vi "ContinousCameraStageV2.vi"() -> ()   [LabVIEW 2016]
uses:
  <vilib>/userdefined/High Color/IMAQdx.ctl
  Controls/0_XYZstage/DoHomeControl.ctl
  Controls/0_XYZstage/JogControlPanel.ctl
  Controls/All_Enums/Enum_TypeDef_JogStepSize.ctl
  Controls/0_XYZstage/CurrentPositionReader.ctl
  Controls/0_XYZstage/BOOLs_AxesEnabled.ctl
  Controls/0_XYZstage/CurrentMonitoring.ctl
  Controls/0_XYZstage/BOOL_Moving.ctl
  Controls/All_Enums/Enum_TypeDef_ImageSharpnessAnalysisMethod.ctl
  Controls/Graph_TypeDef_XY.ctl
  <vilib>/vision/Image Controls.llb/IMAQ Image.ctl
  AerotechLibraries/Motion/MoveIncMultiple.vi
  AerotechLibraries/Motion/WaitMultiple.vi
  <vilib>/vision/driver/NI_Vision_Acquisition_Software.lvlib
  <vilib>/vision/NI_Vision_Development_Module.lvlib
  <vilib>/LabVIEW Interface for Arduino/LabVIEW Interface for Arduino.lvlib
panel:
  out "Z [mm]":dbl
  in  "Tab Control":T1(tab)
  in  "Tab Control 2":enum32{"Stage Controls", "Camera Controls"}(tab)
  in  "Save current position":bool
  in  "Move Stage with Cursors":bool
  in  "Home stage?":T2
  in  "Jogging Controls":T3={"Jog step size"={"X [mm]"=enum."1 mm", "Y [mm]"=enum."1 mm", "Z [mm]"=enum."1 mm"}, "Left"=FALSE, "Right"=FALSE, "Forward"=FALSE, "Backward"=FALSE, "Up"=FALSE, "Down"=FALSE, "Reset position"=FALSE, "Confirm position"=FALSE}
  in  "Axes Speeds":T5={"X [mm/s]"=25.0, "Y [mm/s]"=25.0, "Z [mm/s]"=25.0}
  in  "Move to Absolute Position [mm]":T6
  in  "Move Stage":bool
  out "Cross Point":cluster{"X coordinate":dbl, "Y coordinate":dbl}
  in  "Abort stage":bool
  in  "Tab Control 4":T7(tab)
  in  "Camera Name":T8="cam1" caption="IMAQdx Session"
  in  "Wait time before \nimage capture [s]":dbl=3.5
  in  "Gain of the Camera":dbl(slide) scale=0.0..16.0
  out "Intensity Histogram, current frame":T9(graph)
  in  "Pixel to Micron":dbl=1.5810615417510199 format="%.4f"
  in  "Conversion Method":u16(ring)=1 items=["Strip Centers", "Signal Fit, Left to Right", "Projection + Signal Fit"]
  out "Skew Angle [radians]":dbl format="%.5f"
  out "Skew Angle (uncertainty)":dbl format="%.5f"
  out "um/pixel uncertainty":dbl format="%.4f"
  in  "Strips Coordinates":T6={"X [mm]"=-738.0, "Y [mm]"=-144.0, "Z [mm]"=34.25}
  in  "Strip Pitch (microns)":dbl=74.5 format="%#_13g"
  out "Optimized position":dbl
  out "Uncertainty on position":dbl
  in  "Camera working distance scan":T10={"Stepsize [mm]"=0.2, "Focusing test interval [mm]"=1.5} {"Focusing test interval [mm]" format="%#_13g"}
  in  "Method":T11
  out "Plot":T12
  out "Autofocus Progress":u8(slide) scale=0.0..15.0
  in  "Settings":T13={"Algorithm"=1, "Number of Matches Requested"=1, "Minimum Match Score"=700.0, "SubPixel Accuracy"=TRUE, "Rotation Angle Ranges"=[{"Start"=0.0, "End"=360.0}], "Show Search Area"=FALSE, "Show Result"=TRUE} {"Rotation Angle Ranges"."End" format="%.1f"; "Rotation Angle Ranges"."Start" format="%.1f"; "Minimum Match Score" min=0 max=1000 format="%.2f"; "Number of Matches Requested" min=1; "Algorithm" items=["All", "Low Discrepancy Sampling", "Grayscale Value Pyramid", "Gradients Pyramid"]}
  out "1st Match Distance from Center":cluster{dbl, dbl}
  in  "Template Path":path
  out "1st Matched Position":cluster{"X":dbl, "Y":dbl, "Z [mm]":dbl}
  out "Template Image":T14(plugin-control)
  out "Eccentricity vs. Threshold":cluster{i32[], dbl[]}(graph)
  in  "Threshold Max":sgl=255.0
  in  "Primary Light":bool
  in  "Camera Analysis Function":T15(ring)
  in  "Spotlights":bool
  out "Current stage position":T16
  out "Current monitoring":T17
  out "Homed":bool
  out "Moving":T18
  out "Axis enabled":T19
  out "Wait to capture [ms]":u32=3500
  in  "X [mm]":dbl(slide)=5.417536534446764 scale=-1.0..6.596742723794349 scale format="%#_3g"
  in  "Y [mm]":dbl(slide)=4.6938775510204085 scale=4.720794011715331..-1.0 scale format="%#_3g"
  in  "Tab Control 3":T20(tab)
  out "Current field of view":T14(plugin-control)
  out "Bullseye Out":T14(plugin-control)
  out "Ellipses Out":T14(plugin-control)
  in  "Click to Stop The Program":bool
  out "double( Time, Temp )":dbl[](array[numeric])=[14.0, 16.0, 34.0, 0.8858232498168945, 22.9537926]
  in  "Program Errors 2":errorcluster
  in  "Program Errors":errorcluster
  out "VISA error out":errorcluster
  out "Camera error out":errorcluster
  out "Time and Temperature [*C]":string[](array[string])
  # "CONTINUOUS STAGE AND CAMERA (v2) Brandeis University - Brookhaven National Laboratory * ATLAS Phase II Inner Tracker Upgrade\nPrimary Authors: Prajita Bhattarai (pbhattarai1s@brandeis.edu), Hannah Herde (hherde@brandeis.edu)"
  # "XYZ Stage Performance Monitoring"
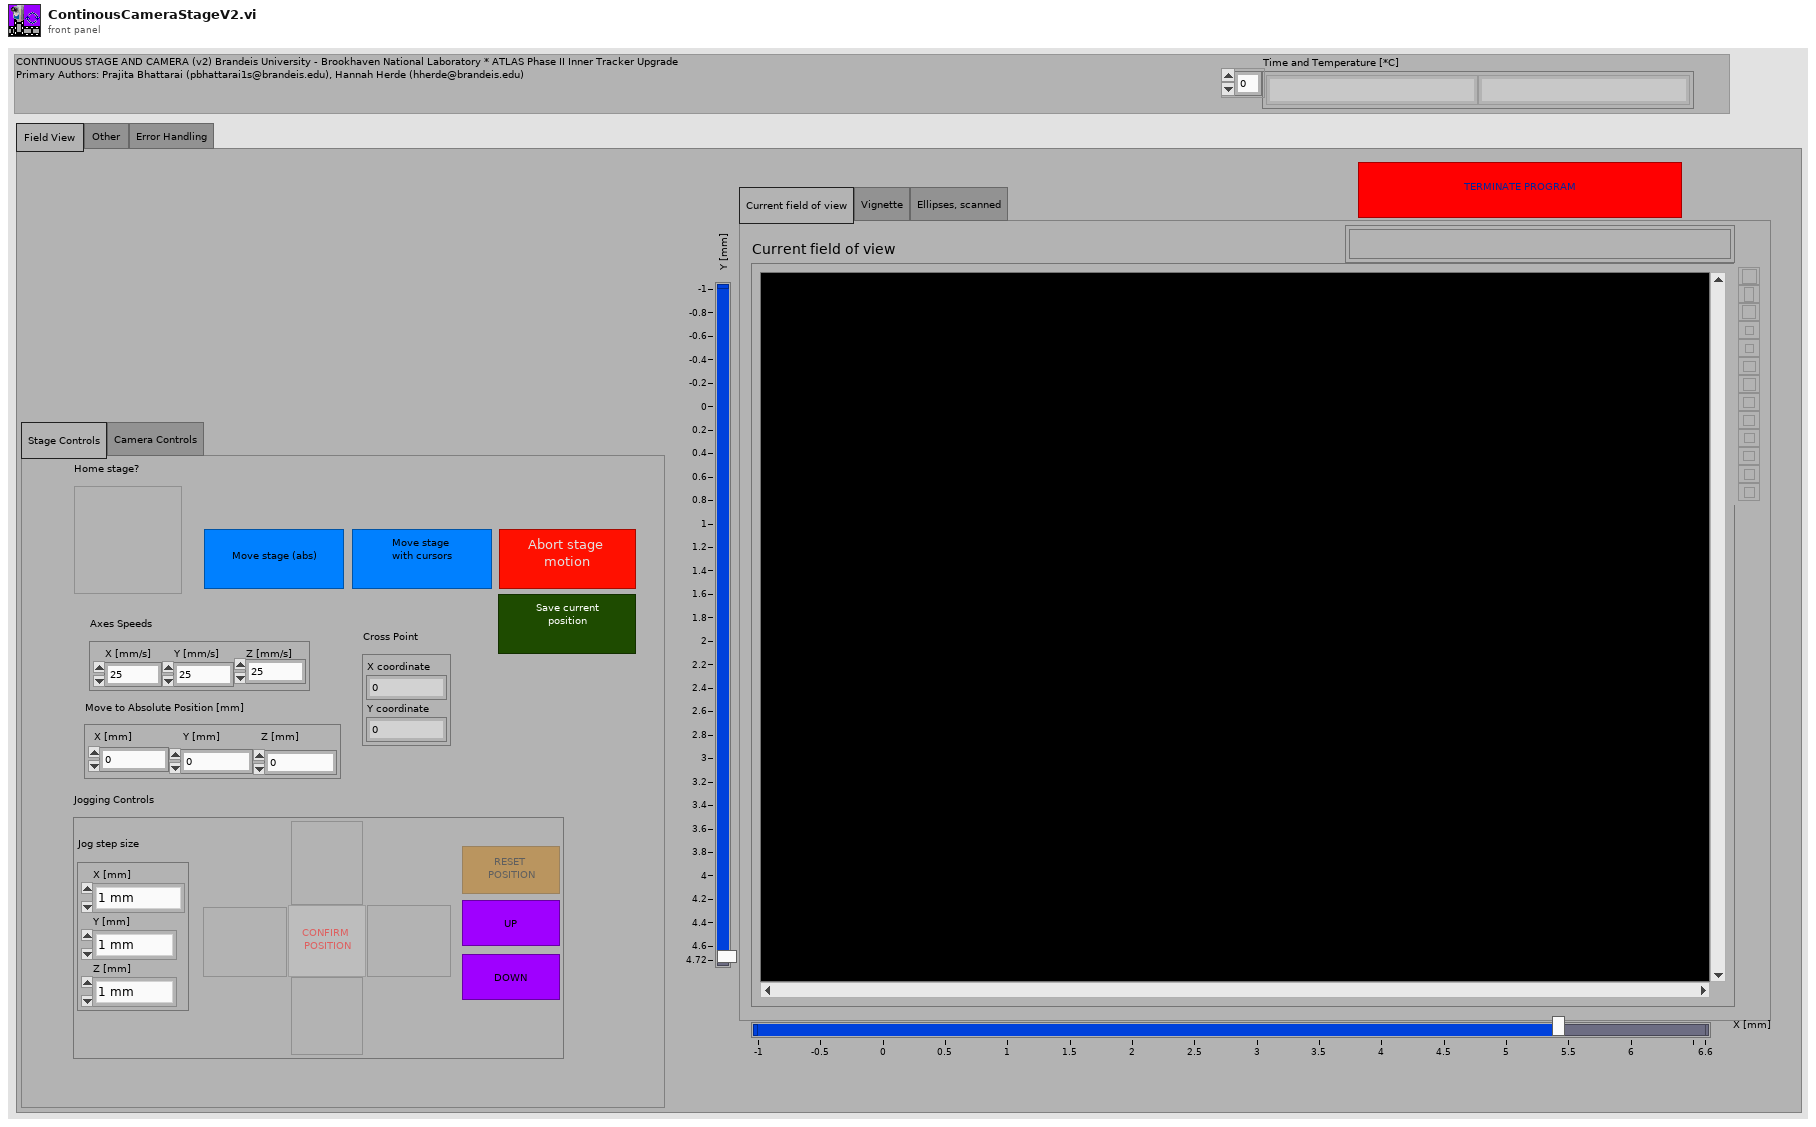
[diagram p1: front panel]
types:
  T1 = enum32{"Field View ", "Other ", "Error Handling"}
  T2 = typedef "DoHomeControl.ctl" = bool
  T3 = typedef "JogControlPanel.ctl" = cluster{"Jog step size":T4, "Left":bool, "Right":bool, "Forward":bool, "Backward":bool, "Up":bool, "Down":bool, "Reset position":bool, "Confirm position":bool}
  T4 = typedef "Enum_TypeDef_JogStepSize.ctl" = cluster{"X [mm]":enum16{"1 um", "5 um", "10 um", "0.1 mm", "0.25 mm", "0.5 mm", "1 mm", "5 mm", "10 mm", "20 mm", "50 mm"}, "Y [mm]":enum16{"1 um", "5 um", "10 um", "0.1 mm", "0.25 mm", "0.5 mm", "1 mm", "5 mm", "10 mm", "20 mm", "50 mm"}, "Z [mm]":enum16{"1 um", "5 um", "10 um", "0.1 mm", "0.25 mm", "0.5 mm", "1 mm", "5 mm", "10 mm", "20 mm", "[None]"}}
  T5 = cluster{"X [mm/s]":dbl, "Y [mm/s]":dbl, "Z [mm/s]":dbl}
  T6 = cluster{"X [mm]":dbl, "Y [mm]":dbl, "Z [mm]":dbl}
  T7 = enum32{"Camera Setup", "Pixel/Micron Conv.", "Height/Autofocus", "Pattern Match", "Vignetting Analysis"}
  T8 = typedef "IMAQdx.ctl" = refnum<k21>
  T9 = cluster{"Starting Value":sgl, "Incremental Value":sgl, "Histogram":u32[]}
  T10 = cluster{"Stepsize [mm]":dbl, "Focusing test interval [mm]":dbl}
  T11 = typedef "Enum_TypeDef_ImageSharpnessAnalysisMethod.ctl" = enum16{"sigma( Intensity )", "Mean( Laplacian Convolution )"}
  T12 = typedef "Graph_TypeDef_XY.ctl" = cluster{"Radius bins":dbl[], "Best Gaussian Fit":dbl[]}[]
  T13 = cluster{"Algorithm":i32, "Number of Matches Requested":i32, "Minimum Match Score":sgl, "SubPixel Accuracy":bool, "Rotation Angle Ranges":cluster{"Start":sgl, "End":sgl}[], "Show Search Area":bool, "Show Result":bool}
  T14 = typedef "IMAQ Image.ctl" = refnum<image>
  T15 = enum16{"[None]", "Determine pixel-micron conversion", "Calibrate camera height", "Find a pattern", "Analyze vignette"}
  T16 = typedef "CurrentPositionReader.ctl" = cluster{"X":dbl, "Y":dbl, "Z":dbl}
  T17 = typedef "CurrentMonitoring.ctl" = cluster{cluster{"X Current Cmd [A]":sgl, "Y Current Cmd [A]":sgl, "Z Current Cmd [A]":sgl}, cluster{"X Current Feedback [A]":sgl, "Y Current Feedback [A]":sgl, "Z Current Feedback [A]":sgl}}
  T18 = typedef "BOOL_Moving.ctl" = bool
  T19 = typedef "BOOLs_AxesEnabled.ctl" = cluster{"X":bool, "Y ":bool, "Z":bool}
  T20 = enum32{"Current field of view", "Vignette", "Ellipses, scanned"}
  T21 = typedef "Image Type" = u32
  T22 = typedef "LabVIEW Interface for Arduino.lvlib/Arduino Resource.ctl" = cluster{"VISA resource":refnum<visa-resource-name>, "Board Type":T23, "Connection Type":enum8{"USB / Serial"}, "Bytes Per Packet (15)":u8}
  T23 = typedef "LabVIEW Interface for Arduino.lvlib/Board Type.ctl" = enum16{"Uno", "Dimuelanove w/Atmega 328", "Mega 2560"}
  T24 = typedef "ArduinoLT-ConfigurationControl.ctl" = cluster{"Lights: Digital I/O Pins":cluster{"Coaxial":u8, "Spotlights":u8}, "Thermistor Settings":cluster{"Analogue Readout Pin":u8, "Vcc Reference Pin":u8, "Paired Resistance (10K Ohms)":dbl, "Units (C)":enum16{"Celsius", "Fahrenheit", "Kelvin"}}}
  T25 = cluster{"Camera session out":T8, "New Image":T14}
  T26 = cluster{"Final X":dbl, "Final Y":dbl, "Final Z":dbl}
  T27 = cluster{"X":dbl, "Y":dbl, "Optimized position":dbl}
  T28 = cluster{"Position":cluster{"x":sgl, "y":sgl}, "Angle":sgl, "Scale":sgl, "Score":sgl, "Bounding Box":cluster{"x":sgl, "y":sgl}[]}[]
  T29 = cluster{"Matches (pixel)[0]":cluster{"Position":cluster{"x":sgl, "y":sgl}, "Angle":sgl, "Scale":sgl, "Score":sgl, "Bounding Box":cluster{"x":sgl, "y":sgl}[]}, "Matches (pixel)[1]":cluster{"Position":cluster{"x":sgl, "y":sgl}, "Angle":sgl, "Scale":sgl, "Score":sgl, "Bounding Box":cluster{"x":sgl, "y":sgl}[]}, "Matches (pixel)[2]":cluster{"Position":cluster{"x":sgl, "y":sgl}, "Angle":sgl, "Scale":sgl, "Score":sgl, "Bounding Box":cluster{"x":sgl, "y":sgl}[]}, "Matches (pixel)[3]":cluster{"Position":cluster{"x":sgl, "y":sgl}, "Angle":sgl, "Scale":sgl, "Score":sgl, "Bounding Box":cluster{"x":sgl, "y":sgl}[]}, "Matches (pixel)[4]":cluster{"Position":cluster{"x":sgl, "y":sgl}, "Angle":sgl, "Scale":sgl, "Score":sgl, "Bounding Box":cluster{"x":sgl, "y":sgl}[]}, "Matches (pixel)[5]":cluster{"Position":cluster{"x":sgl, "y":sgl}, "Angle":sgl, "Scale":sgl, "Score":sgl, "Bounding Box":cluster{"x":sgl, "y":sgl}[]}, "Matches (pixel)[6]":cluster{"Position":cluster{"x":sgl, "y":sgl}, "Angle":sgl, "Scale":sgl, "Score":sgl, "Bounding Box":cluster{"x":sgl, "y":sgl}[]}, "Matches (pixel)[7]":cluster{"Position":cluster{"x":sgl, "y":sgl}, "Angle":sgl, "Scale":sgl, "Score":sgl, "Bounding Box":cluster{"x":sgl, "y":sgl}[]}, "Matches (pixel)[8]":cluster{"Position":cluster{"x":sgl, "y":sgl}, "Angle":sgl, "Scale":sgl, "Score":sgl, "Bounding Box":cluster{"x":sgl, "y":sgl}[]}}
  T30 = cluster{"Position":cluster{"x":sgl, "y":sgl}, "Angle":sgl, "Scale":sgl, "Score":sgl, "Bounding Box":cluster{"x":sgl, "y":sgl}[]}
  T31 = cluster{cluster{"X Current Cmd [A]":sgl, "Y Current Cmd [A]":sgl, "Z Current Cmd [A]":sgl}, cluster{"X Current Feedback [A]":sgl, "Y Current Feedback [A]":sgl, "Z Current Feedback [A]":sgl}}
  T32 = cluster{"Step size [mm]":dbl, "Step size [mm]":dbl, "Step size [mm]":dbl}
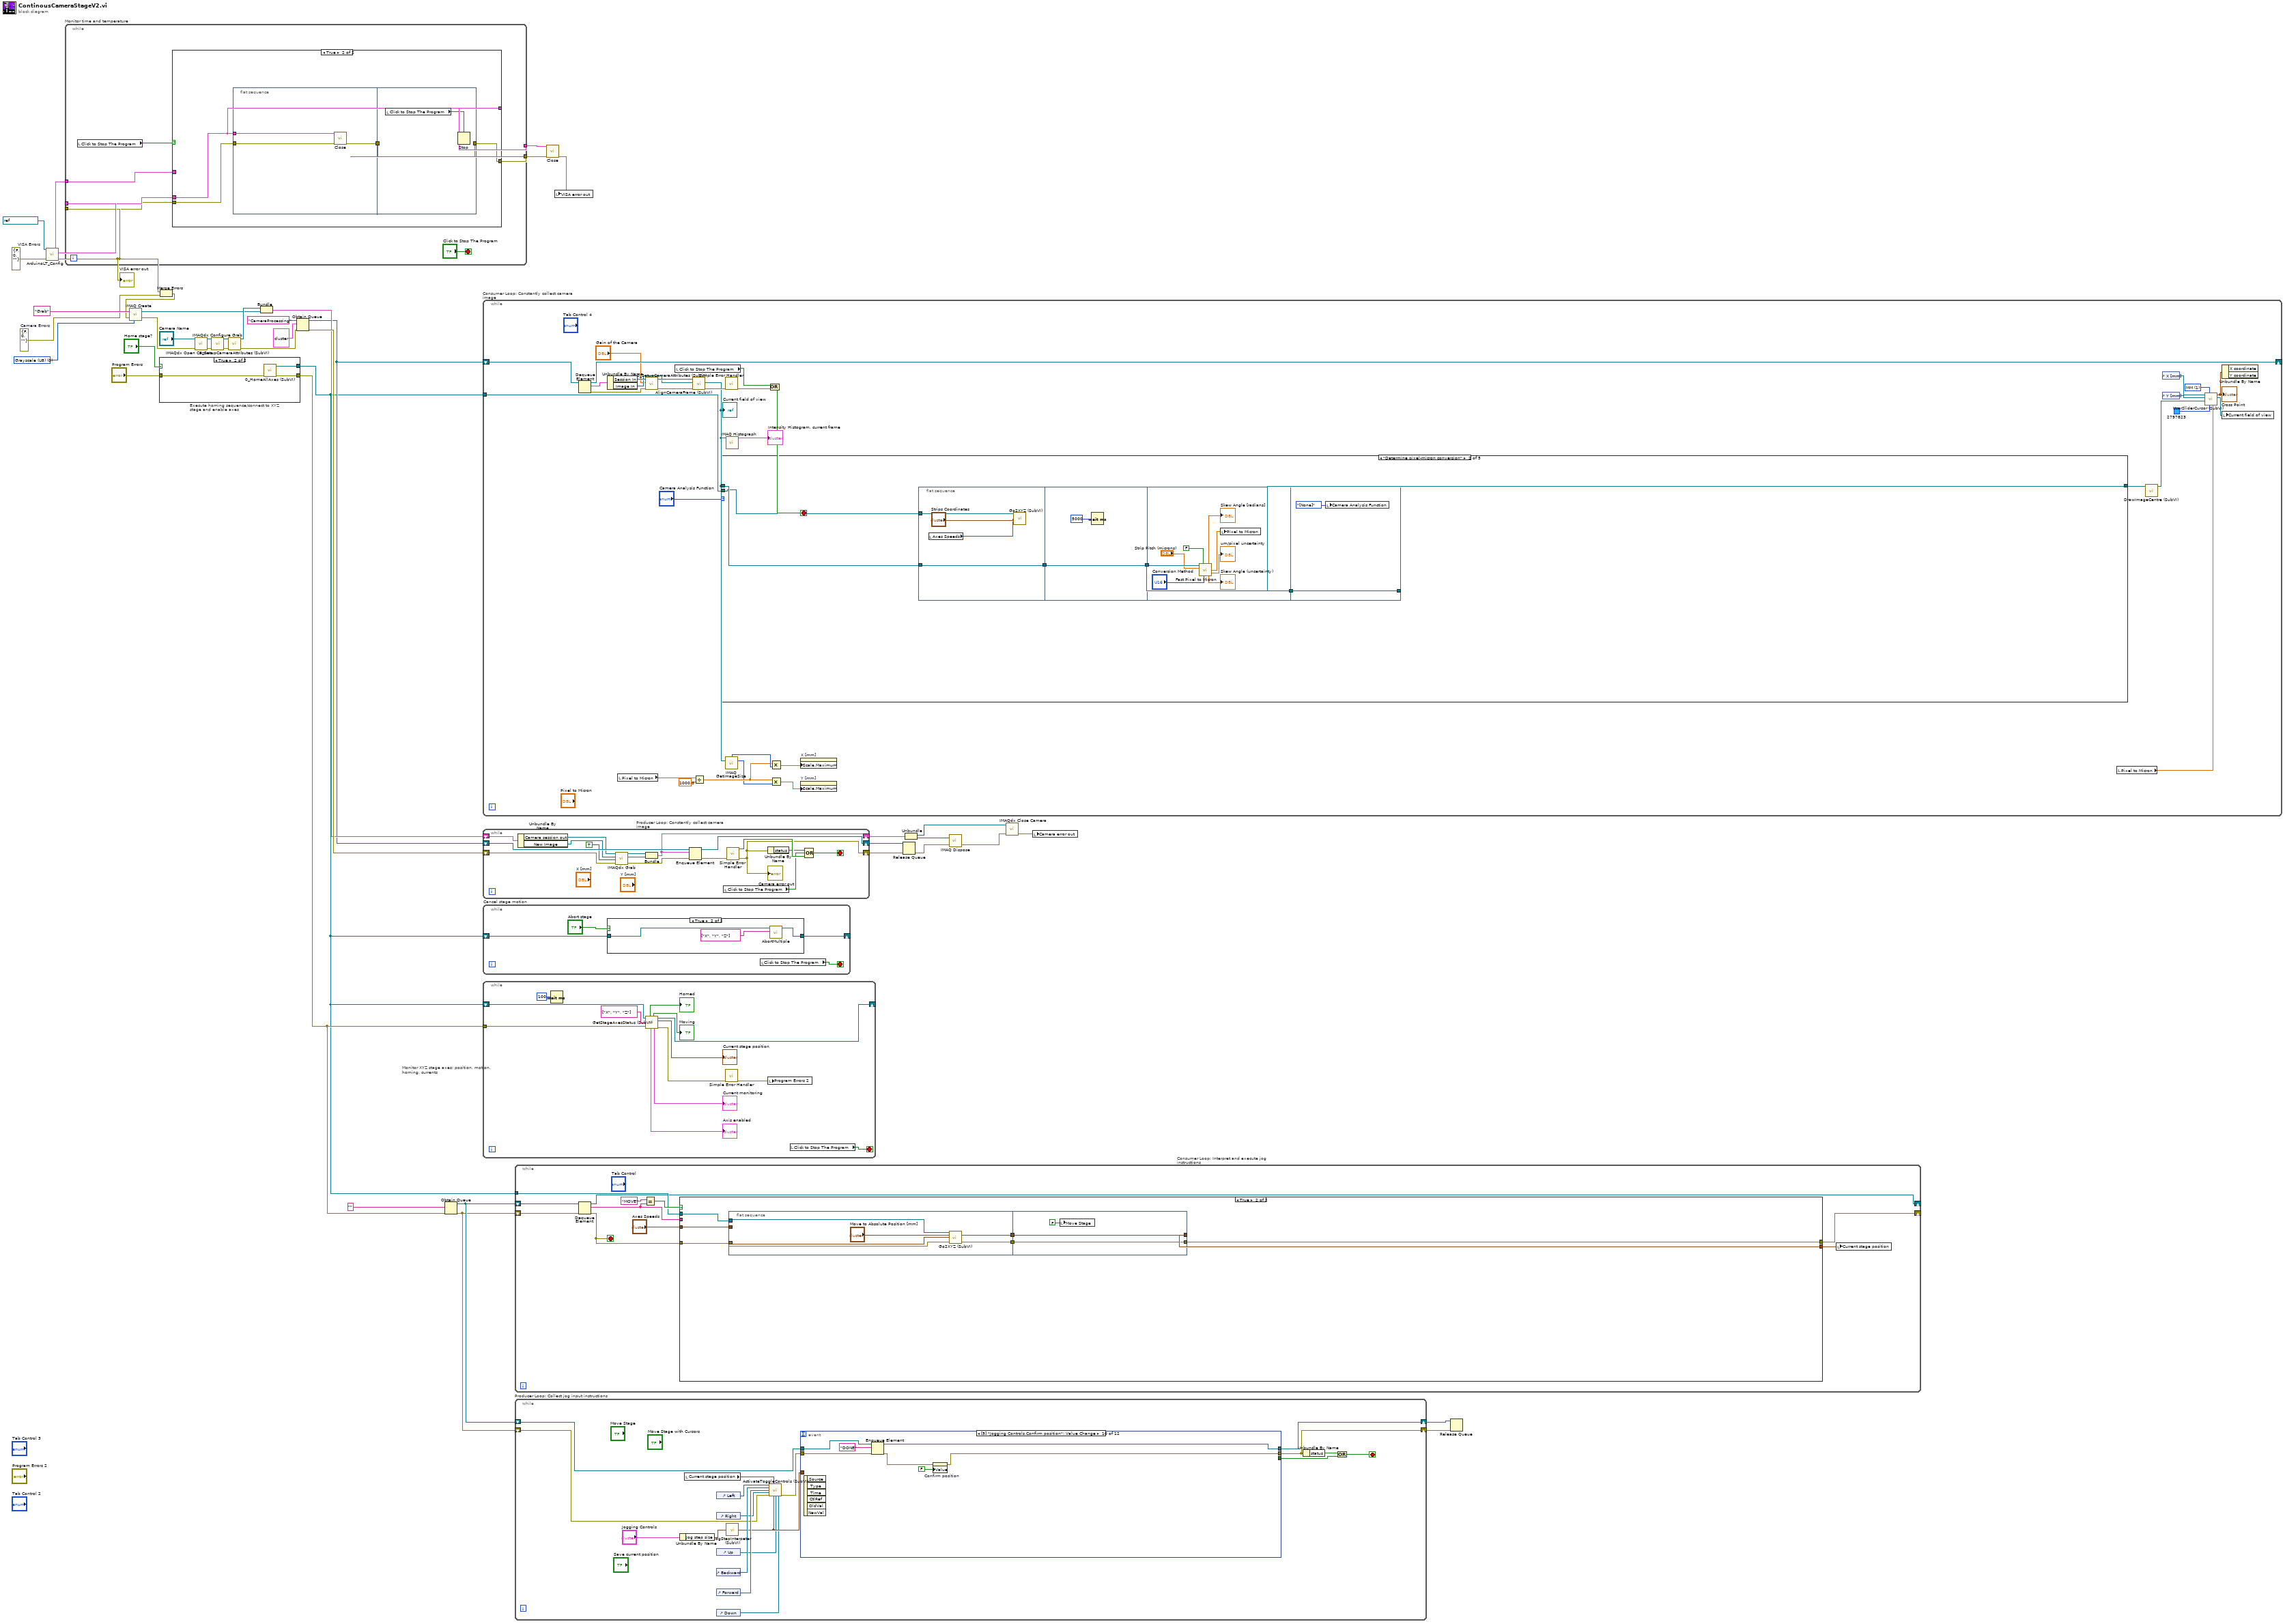
[diagram p0: block diagram]
diagram:
  w9 = errorcluster {"status"=FALSE, "code"=0, "source"=""}  # VISA Errors
  w2 = errorcluster {"status"=FALSE, "code"=0, "source"=""}  # Camera Errors
  w41 = T21 0 items=["Grayscale (U8)", "Grayscale (I16)", "Grayscale (SGL)", "Complex (CSG)", "RGB (U32)", "HSL (U32)", "RGB (U64)", "Grayscale (U16)"] ("Image Type")
  n1 = call "ArduinoLT_Config.vi"("error in"=w9, "VISA resource"=refnum<visa-resource-name> "LightsCTRL") -> ("error out"=w3:errorcluster, "Arduino Resource"=w7:T22, "Arduino Configuration OUT"=w8:T24)  [unwired: 3 in, 1 out]
  "VISA error out" <- w3
  n2 = while "Monitor time and temperature" {
    tunnel: w3 -> [w47]
    tunnel: w8 -> [w49]
    tunnel: w7 -> [w48]
    tunnel: [w46] -> w6
    tunnel: [w45] -> w4
    stop <- "Click to Stop The Program" stop-if-true
    n3 = local read "Click to Stop The Program"() -> (w44:bool)
    n4 = case shown="True" w44 {
      tunnel: w49 -> [w59 _]
      tunnel: w48 -> [w58 w66]
      tunnel: w47 -> [w57 w69]
      tunnel: [w56 w66] -> w46
      tunnel: [w52 w68] -> w45
      frame False {
        n5 = Wait (ms)(milliseconds to wait=u32 1000) -> ()  [unwired: 1 out]
        n6 = call "ArduinoLT_Collect_Control.vi"("Arduino Configuration"=w59, "error in"=w57, "Arduino Resource IN"=w58, "Spotlights"="Spotlights", "Coaxial light"="Primary Light") -> ("error out"=w51:errorcluster, "Arduino Resource OUT"=w56:T22, "Thermometer [C]"=w55:dbl)  [unwired: 4 in]
        n7 = local write "VISA error out"(w51) -> ()
        n8 = Multiply(x="Wait time before \nimage capture [s]", y=u32 1000) -> (x*y=→"Wait to capture [ms]":dbl)
        n9 = call "ArduinoLT-TimeAndTempature.vi"("error in (no error)"=w51, "Temperature"=w55) -> ("error out"=w52:errorcluster, "double( Time, Temp )"=→"double( Time, Temp )":dbl[], "str( Time, Temp )"=→"Time and Temperature [*C]":string[])  [unwired: 7 in]
        n10 = local write "VISA error out"(w52) -> ()
      }
      frame True {
        n11 = flat-sequence {
          tunnel: w66 -> [w72]
          tunnel: w69 -> [w71]
          tunnel: [w70] -> w67
          tunnel: [w74] -> w68
          tunnel: w67 -> [w74]
          frame #0 {
            n12 = call <vilib>:"Close.vi"("Arduino Resource"=w72, "error in"=w71) -> ("error out"=w70:errorcluster)  [unwired: 13 in]
          }
          frame #1 {
            n13 = local read "Click to Stop The Program"() -> (w73:bool)
            n14 = Stop(stop? (T)=w73) -> ()
          }
        }
      }
    }
  }
  n15 = case "Execute homing sequence/connect to XYZ stage and enable axes" shown="True" "Home stage?" {
    tunnel: [w77 w83] -> w12
    tunnel: "Program Errors" -> [w75 w81]
    tunnel: [w76 w82] -> w11
    frame False {
      n16 = call "Connect.vi"("error in (no error)"=w75) -> ("error out"=w80:errorcluster, "controller"=w79:refnum<k24>)  [unwired: 9 in]
      n17 = call "EnableMultiple.vi"("error in (no error)"=w80, "axis names"=string[] ["X", "Y", "Z"] ("Axes Names"), "controller in"=w79) -> ("error out"=w77:errorcluster, "controller out"=w76:refnum<k24>)  [unwired: 7 in]
    }
    frame True {
      n18 = call "0_HomeAllAxes (SubVI).vi"("error in (no error)"=w81) -> ("error out"=w83:errorcluster, "controller out"=w82:refnum<k24>)  [unwired: 7 in, 2 out]
    }
  }
  n19 = Merge Errors(w3, w2) -> (w1:errorcluster)
  n20 = call "IMAQ Create"("Image Name"="Grab", "Image Type"=w41, "error in (no error)"=w1) -> ("New Image"=w30:T14, "error out"=w38:errorcluster)  [unwired: 1 in, 1 out]
  n21 = call <vilib>:"IMAQdx Open Camera.vi"("error in"=w38, "Session In"="Camera Name") -> ("error out"=w39:errorcluster, "Session Out"=w42:T8)  [unwired: 1 in, 7 out]
  n22 = call <vilib>:"IMAQdx Configure Grab.vi"("error in"=w39, "Session In"=w42) -> ("error out"=w34:errorcluster, "Session Out"=w35:T8)  [unwired: 8 out]
  n23 = call "0_SetupCameraAttributes (SubVI).vi"("error in (no error)"=w34, "Camera session in"=w35) -> ("error out"=w33:errorcluster, "Camera session out"=w31:T8)  [unwired: 8 in]
  n24 = Bundle("Camera session out"=w31, "New Image"=w30) -> (w29:T25)  [unwired: 1 in]
  n25 = Obtain Queue(name (unnamed)="CameraProcessing", element data type=cluster{"Session In":T8, "Image In":T14} {"Session In"="", "Image In"=refnum}, error in (no error)=w33) -> (queue out=w21:refnum<queue>, error out=w32:errorcluster)  [unwired: 2 in, 1 out]
  n26 = Obtain Queue(element data type="", error in (no error)=w12) -> (queue out=w16:refnum<queue>, error out=w15:errorcluster)  [unwired: 3 in, 1 out]
  n27 = while "Consumer Loop: Constantly collect camera image" {
    shift-right: [w112] -> _
    shift-left: w21 -> [w116]
    tunnel: w11 -> [w99]
    stop <- w114 stop-if-true
    w89 = u16 1 items=["MM"=1, "Pixel"=0] ("Coordinates Unit")
    n28 = Dequeue Element(queue=w116) -> (queue out=w112:refnum<queue>, element=w115:cluster{"Session In":T8, "Image In":T14}, error out=w113:errorcluster)  [unwired: 2 in, 1 out]
    n29 = Unbundle By Name(w115) -> ("Session In"=w111:T8, "Image In"=w109:T14)
    n30 = local read "Pixel to Micron"() -> (w96:dbl)
    n31 = call "0_SetupCameraAttributes (SubVI).vi"("error in (no error)"=w113, "Gain"="Gain of the Camera", "Camera session in"=w111) -> ("error out"=w108:errorcluster, "Camera session out"=w110:T8)  [unwired: 7 in]
    n32 = local read "Click to Stop The Program"() -> (w105:bool)
    n33 = call "AlignCameraFrame (SubVI).vi"("error in (no error)"=w108, "Image Src"=w109, "Camera session in"=w110) -> ("error out"=w107:errorcluster, "Image Dst Out"=w86:T14)  [unwired: 6 in, 1 out]
    "Current field of view" <- w86
    n34 = Divide(x=w96, y=1000.0) -> (x/y=w93:dbl)
    n35 = case shown="\"Determine pixel-micron conversion\"" "Camera Analysis Function" {
      tunnel: w86 -> [w117 w122 w141 w240 w252]
      tunnel: [w117 w121 w140 w211 w251] -> w87
      tunnel: w99 -> [_ w120 w142 _ _]
      frame "[None]", Default {
        # "Do nothing"
      }
      frame "Determine pixel-micron conversion" {
        n36 = flat-sequence {
          tunnel: w122 -> [w127]
          tunnel: [w127] -> w119
          tunnel: w120 -> [w125]
          tunnel: w119 -> [w129]
          tunnel: [w129] -> w118
          tunnel: [w136] -> w123
          tunnel: w118 -> [w136]
          tunnel: [w139] -> w121
          tunnel: w123 -> [w139]
          frame #0 {
            n37 = local read "Axes Speeds"() -> (w124:T5)
            n38 = call "Go2XYZ (SubVI).vi"(".NET Refnum in"=w125, "Go to Coordinates"="Strips Coordinates", "Axis Speeds"=w124) -> ()  [unwired: 8 in, 5 out]
          }
          frame #1 {
            n39 = Wait (ms)(milliseconds to wait=u32 5000) -> ()  [unwired: 1 out]
          }
          frame #2 {
            n40 = call "Fast Pixel to Micron.vi"("Refnum In"=w136, "Absolute Constraints"=FALSE ("Apply absolute constraints?"), "Strip Pitch (microns)"="Strip Pitch (microns)", "Conversion Method"="Conversion Method") -> ("FFT Angle (Rad)"=→"Skew Angle [radians]":dbl, "Microns/Pixel (Corrected)"=w135:dbl, "Error (Corrected)"=→"um/pixel uncertainty":dbl, "FFT Error (Rad)"=→"Skew Angle (uncertainty)":dbl)  [unwired: 5 in, 3 out]
            n41 = local write "Pixel to Micron"(w135) -> ()
          }
          frame #3 {
            n42 = local write "Camera Analysis Function"(T15."[None]" ("Camera Analysis Function")) -> ()
          }
        }
      }
      frame "Calibrate camera height" {
        n43 = flat-sequence {
          tunnel: w141 -> [w161]
          tunnel: w142 -> [w150]
          tunnel: [w160] -> w148
          tunnel: [w150] -> w147
          tunnel: w148 -> [w189]
          tunnel: [w189] -> w146
          tunnel: [w188] -> w145
          tunnel: w147 -> [w188]
          tunnel: [w187] -> w144
          tunnel: w146 -> [w198]
          tunnel: [w198] -> w143
          tunnel: w145 -> [w193]
          tunnel: w144 -> [w190]
          tunnel: w143 -> [w208]
          tunnel: [w208] -> w140
          frame #0 {
            n44 = Unbundle By Name("Camera working distance scan") -> ("Stepsize [mm]"=w163:dbl, "Focusing test interval [mm]"=w162:dbl)
            n45 = Multiply(x=w162, y=2.0) -> (x*y=w164:dbl)
            n46 = local read "Current stage position"() -> (w152:T16)
            n47 = Divide(x=w164, y=w163) -> (x/y=w149:dbl)
            n48 = for {
              N: w149 -> [_]
              tunnel: w152 -> [w186]
              tunnel: w163 -> [w183]
              tunnel: w162 -> [w179]
              tunnel: w161 -> [w178]
              tunnel: [w177] -> w160
              tunnel: w150 -> [w176]
              tunnel: [w172] -> w158 mode=indexing
              tunnel: [w170] -> w154 mode=indexing
              tunnel: [w169] -> w159 mode=indexing
              i -> [w168]
              n49 = Unbundle By Name(w186) -> ("X"=w185:dbl, "Y"=w184:dbl, "Z"=w182:dbl)
              n50 = Multiply(x=w183, y=w168) -> (x*y=w180:dbl)
              n51 = Subtract(x=w182, y=w179) -> (x-y=w181:dbl)
              n52 = Increment(x=w168) -> (x+1=→"Autofocus Progress":i32)
              n53 = Add(x=w181, y=w180) -> (x+y=w169:dbl)
              n54 = local read "Axes Speeds"() -> (w174:T5)
              n55 = Bundle("X"=w185, "Y"=w184, w169) -> (w175:cluster{"X":dbl, "Y":dbl, dbl})  [unwired: 1 in]
              n56 = call "Go2XYZwWait (SubVI).vi"(".NET Refnum in"=w176, "Go to Coordinates"=w175, "Axis Speeds"=w174) -> ("Final Position"=w171:T26)  [unwired: 8 in, 4 out]
              n57 = local write "Current stage position"(w171) -> ()
              n58 = call "MeasureImageSharpness.vi"("Method"="Method", "Image In"=w178) -> ("Sharpness Uncertainty"=w170:dbl, "Sharpness"=w172:dbl, "Image Out"=w177:T14)  [unwired: 6 in, 1 out]
            }
            n59 = property on="Autofocus Progress" class="Slide (strict)"("Scale.Maximum"=w149) -> ()  [unwired: 2 in, 2 out]
            n60 = Unbundle By Name(w152) -> ("Z"=→"Z [mm]":dbl)  [unwired: 2 out]
            n61 = local write "Current field of view"(w160) -> ()
            n62 = call "FitGaussian3(SubVI).vi"("x values"=w159, "y values"=w158, "delta y values"=w154, "confidence level"=0.68) -> ("Plot"=→"Plot":T12, "Optimized position"=→"Optimized position":dbl, "Uncertainty on position"=→"Uncertainty on position":dbl)  [unwired: 10 in, 3 out]
          }
          frame #1 {
            n63 = call "Optimal Height?"() -> ("Yes"=w187:bool)  [unwired: 16 in, 3 out]
          }
          frame #2 {
            n64 = local read "Current stage position"() -> (w195:T16)
            n65 = Unbundle By Name(w195) -> ("X"=w196:dbl, "Y"=w197:dbl)  [unwired: 1 out]
            n66 = case shown="False" w190 {
              tunnel: w196 -> [w202 w206]
              tunnel: w197 -> [w201 w205]
              tunnel: [w199 w203] -> w194
              frame False {
                n67 = local read "Z [mm]"() -> (w200:dbl)
                n68 = Bundle("X"=w202, "Y"=w201, "Z [mm]"=w200) -> (w199:cluster{"X":dbl, "Y":dbl, "Z [mm]":dbl})  [unwired: 1 in]
              }
              frame True {
                n69 = local read "Optimized position"() -> (w204:dbl)
                n70 = Bundle("X"=w206, "Y"=w205, "Optimized position"=w204) -> (w203:T27)  [unwired: 1 in]
              }
            }
            n71 = local read "Axes Speeds"() -> (w192:T5)
            n72 = call "Go2XYZ (SubVI).vi"(".NET Refnum in"=w193, "Go to Coordinates"=w194, "Axis Speeds"=w192) -> ("Final Position"=w191:T26)  [unwired: 8 in, 4 out]
            n73 = local write "Current stage position"(w191) -> ()
          }
          frame #3 {
            n74 = local write "Camera Analysis Function"(T15."[None]" ("Camera Analysis Function")) -> ()
          }
        }
      }
      frame "Find a pattern" {
        w227 = 2 ("y")